vi "FlexMag - 24-03-2023.vi"() -> ()   [LabVIEW 2018] (continued)
                }
              }
              frame True {
                n6892 = stacked-sequence {
                  tunnel: w12617 -> [_ w12620]
                  frame #0 {
                    n6893 = local write "current step"(6.0 ("y")) -> ()
                  }
                  frame #1 {
                    n6894 = Subtract(x=w12620, y=5.0) -> (x-y=w12621:dbl)
                    n6895 = local write "step count"(w12621) -> ()
                  }
                }
              }
            }
            n6896 = local write "QR off mode"(TRUE ("QR manual mode")) -> ()
          }
          frame #1 {
            n6897 = local read "qr wait second"() -> (w12622:u32)
            n6898 = Multiply(x=u32 1000 ("milliseconds to wait"), y=w12622) -> (x*y=w12623:u32)
            n6899 = Wait (ms)(milliseconds to wait=w12623) -> ()  [unwired: 1 out]
          }
          frame #2 {
            n6900 = disable-structure shown="Disabled" {
              frame Disabled {
                n6901 = local write "Interrupt DI"(TRUE ("Interrupt DI")) -> ()
                n6902 = Wait (ms)(milliseconds to wait=u32 100) -> ()  [unwired: 1 out]
              }
              frame Enabled {
              }
            }
          }
          frame #3 {
            n6903 = local read "step count"() -> (w12628:dbl)
            n6904 = Greater?(x=w12628, y=0.0) -> (0:w12629:bool)
            n6905 = case shown="True" w12629 {
              frame False {
              }
              frame True {
                n6906 = local write "QR continuous mode"(TRUE ("QR continuous mode")) -> ()
              }
            }
          }
        }
      }
      frame 7 {
        # "barcode 6"
        n6907 = stacked-sequence {
          frame #0 {
            n6908 = local read "forward roll"() -> (w12633:bool)
            n6909 = local read "step count 2"() -> (w12631:dbl)
            n6910 = local read "back roll"() -> (w12632:bool)
            n6911 = Wait (ms)(milliseconds to wait=u32 100) -> ()  [unwired: 1 out]
            n6912 = case shown="False" w12633 {
              tunnel: w12632 -> [w12636 _]
              tunnel: w12631 -> [_ w12639]
              frame False {
                n6913 = case shown="True" w12636 {
                  frame False {
                  }
                  frame True {
                    n6914 = stacked-sequence {
                      frame #0 {
                        n6915 = local write "current step"(6.0 ("current step")) -> ()
                      }
                      frame #1 {
                        n6916 = local write "step count"(6.0 ("y")) -> ()
                      }
                    }
                  }
                }
              }
              frame True {
                n6917 = stacked-sequence {
                  tunnel: w12639 -> [_ w12642]
                  frame #0 {
                    n6918 = local write "current step"(7.0 ("y")) -> ()
                  }
                  frame #1 {
                    n6919 = Subtract(x=w12642, y=6.0) -> (x-y=w12643:dbl)
                    n6920 = local write "step count"(w12643) -> ()
                  }
                }
              }
            }
            n6921 = local write "QR off mode"(TRUE ("QR manual mode")) -> ()
          }
          frame #1 {
            n6922 = local read "qr wait second"() -> (w12644:u32)
            n6923 = Multiply(x=u32 1000 ("milliseconds to wait"), y=w12644) -> (x*y=w12645:u32)
            n6924 = Wait (ms)(milliseconds to wait=w12645) -> ()  [unwired: 1 out]
          }
          frame #2 {
            n6925 = disable-structure shown="Disabled" {
              frame Disabled {
                n6926 = local write "Interrupt DI"(TRUE ("Interrupt DI")) -> ()
                n6927 = Wait (ms)(milliseconds to wait=u32 100) -> ()  [unwired: 1 out]
              }
              frame Enabled {
              }
            }
          }
          frame #3 {
            n6928 = local read "step count"() -> (w12650:dbl)
            n6929 = Greater?(x=w12650, y=0.0) -> (0:w12651:bool)
            n6930 = case shown="True" w12651 {
              frame False {
              }
              frame True {
                n6931 = local write "QR continuous mode"(TRUE ("QR continuous mode")) -> ()
              }
            }
          }
        }
      }
      frame 8 {
        # "barcode 7"
        n6932 = stacked-sequence {
          frame #0 {
            n6933 = local read "forward roll"() -> (w12655:bool)
            n6934 = local read "step count 2"() -> (w12653:dbl)
            n6935 = local read "back roll"() -> (w12654:bool)
            n6936 = Wait (ms)(milliseconds to wait=u32 100) -> ()  [unwired: 1 out]
            n6937 = case shown="True" w12655 {
              tunnel: w12654 -> [w12658 _]
              tunnel: w12653 -> [_ w12661]
              frame False {
                n6938 = case shown="True" w12658 {
                  frame False {
                  }
                  frame True {
                    n6939 = stacked-sequence {
                      frame #0 {
                        n6940 = local write "current step"(7.0 ("current step")) -> ()
                      }
                      frame #1 {
                        n6941 = local write "step count"(7.0 ("y")) -> ()
                      }
                    }
                  }
                }
              }
              frame True {
                n6942 = stacked-sequence {
                  tunnel: w12661 -> [_ w12664]
                  frame #0 {
                    n6943 = local write "current step"(8.0 ("y")) -> ()
                  }
                  frame #1 {
                    n6944 = Subtract(x=w12664, y=7.0) -> (x-y=w12665:dbl)
                    n6945 = local write "step count"(w12665) -> ()
                  }
                }
              }
            }
            n6946 = local write "QR off mode"(TRUE ("QR manual mode")) -> ()
          }
          frame #1 {
            n6947 = local read "qr wait second"() -> (w12666:u32)
            n6948 = Multiply(x=u32 1000 ("milliseconds to wait"), y=w12666) -> (x*y=w12667:u32)
            n6949 = Wait (ms)(milliseconds to wait=w12667) -> ()  [unwired: 1 out]
          }
          frame #2 {
            n6950 = disable-structure shown="Disabled" {
              frame Disabled {
                n6951 = local write "Interrupt DI"(TRUE ("Interrupt DI")) -> ()
                n6952 = Wait (ms)(milliseconds to wait=u32 100) -> ()  [unwired: 1 out]
              }
              frame Enabled {
              }
            }
          }
          frame #3 {
            n6953 = local read "step count"() -> (w12672:dbl)
            n6954 = Greater?(x=w12672, y=0.0) -> (0:w12673:bool)
            n6955 = case shown="True" w12673 {
              frame False {
              }
              frame True {
                n6956 = local write "QR continuous mode"(TRUE ("QR continuous mode")) -> ()
              }
            }
          }
        }
      }
      frame 9 {
        # "barcode 8"
        n6957 = stacked-sequence {
          frame #0 {
            n6958 = local read "forward roll"() -> (w12677:bool)
            n6959 = local read "step count 2"() -> (w12675:dbl)
            n6960 = local read "back roll"() -> (w12676:bool)
            n6961 = Wait (ms)(milliseconds to wait=u32 100) -> ()  [unwired: 1 out]
            n6962 = case shown="False" w12677 {
              tunnel: w12676 -> [w12680 _]
              tunnel: w12675 -> [_ w12683]
              frame False {
                n6963 = case shown="True" w12680 {
                  frame False {
                  }
                  frame True {
                    n6964 = stacked-sequence {
                      frame #0 {
                        n6965 = local write "current step"(8.0 ("current step")) -> ()
                      }
                      frame #1 {
                        n6966 = local write "step count"(8.0 ("y")) -> ()
                      }
                    }
                  }
                }
              }
              frame True {
                n6967 = stacked-sequence {
                  tunnel: w12683 -> [_ w12686]
                  frame #0 {
                    n6968 = local write "current step"(9.0 ("y")) -> ()
                  }
                  frame #1 {
                    n6969 = Subtract(x=w12686, y=8.0) -> (x-y=w12687:dbl)
                    n6970 = local write "step count"(w12687) -> ()
                  }
                }
              }
            }
            n6971 = local write "QR off mode"(TRUE ("QR manual mode")) -> ()
          }
          frame #1 {
            n6972 = local read "qr wait second"() -> (w12688:u32)
            n6973 = Multiply(x=u32 1000 ("milliseconds to wait"), y=w12688) -> (x*y=w12689:u32)
            n6974 = Wait (ms)(milliseconds to wait=w12689) -> ()  [unwired: 1 out]
          }
          frame #2 {
            n6975 = disable-structure shown="Disabled" {
              frame Disabled {
                n6976 = local write "Interrupt DI"(TRUE ("Interrupt DI")) -> ()
                n6977 = Wait (ms)(milliseconds to wait=u32 100) -> ()  [unwired: 1 out]
              }
              frame Enabled {
              }
            }
          }
          frame #3 {
            n6978 = local read "step count"() -> (w12694:dbl)
            n6979 = Greater?(x=w12694, y=0.0) -> (0:w12695:bool)
            n6980 = case shown="True" w12695 {
              frame False {
              }
              frame True {
                n6981 = local write "QR continuous mode"(TRUE ("QR continuous mode")) -> ()
              }
            }
          }
        }
      }
      frame 10 {
        # "barcode 9"
        n6982 = stacked-sequence {
          frame #0 {
            n6983 = local read "forward roll"() -> (w12699:bool)
            n6984 = local read "step count 2"() -> (w12697:dbl)
            n6985 = local read "back roll"() -> (w12698:bool)
            n6986 = Wait (ms)(milliseconds to wait=u32 100) -> ()  [unwired: 1 out]
            n6987 = case shown="True" w12699 {
              tunnel: w12698 -> [w12702 _]
              tunnel: w12697 -> [_ w12705]
              frame False {
                n6988 = case shown="True" w12702 {
                  frame False {
                  }
                  frame True {
                    n6989 = stacked-sequence {
                      frame #0 {
                        n6990 = local write "current step"(9.0 ("current step")) -> ()
                      }
                      frame #1 {
                        n6991 = local write "step count"(9.0 ("y")) -> ()
                      }
                    }
                  }
                }
              }
              frame True {
                n6992 = stacked-sequence {
                  tunnel: w12705 -> [_ w12708]
                  frame #0 {
                    n6993 = local write "current step"(10.0 ("y")) -> ()
                  }
                  frame #1 {
                    n6994 = Subtract(x=w12708, y=9.0) -> (x-y=w12709:dbl)
                    n6995 = local write "step count"(w12709) -> ()
                  }
                }
              }
            }
            n6996 = local write "QR off mode"(TRUE ("QR manual mode")) -> ()
          }
          frame #1 {
            n6997 = local read "qr wait second"() -> (w12710:u32)
            n6998 = Multiply(x=u32 1000 ("milliseconds to wait"), y=w12710) -> (x*y=w12711:u32)
            n6999 = Wait (ms)(milliseconds to wait=w12711) -> ()  [unwired: 1 out]
          }
          frame #2 {
            n7000 = disable-structure shown="Disabled" {
              frame Disabled {
                n7001 = local write "Interrupt DI"(TRUE ("Interrupt DI")) -> ()
                n7002 = Wait (ms)(milliseconds to wait=u32 100) -> ()  [unwired: 1 out]
              }
              frame Enabled {
              }
            }
          }
          frame #3 {
            n7003 = local read "step count"() -> (w12716:dbl)
            n7004 = Greater?(x=w12716, y=0.0) -> (0:w12717:bool)
            n7005 = case shown="True" w12717 {
              frame False {
              }
              frame True {
                n7006 = local write "QR continuous mode"(TRUE ("QR continuous mode")) -> ()
              }
            }
          }
        }
      }
      frame 11 {
        # "barcode 10"
        n7007 = stacked-sequence {
          frame #0 {
            n7008 = local read "forward roll"() -> (w12721:bool)
            n7009 = local read "step count 2"() -> (w12719:dbl)
            n7010 = local read "back roll"() -> (w12720:bool)
            n7011 = Wait (ms)(milliseconds to wait=u32 100) -> ()  [unwired: 1 out]
            n7012 = case shown="False" w12721 {
              tunnel: w12720 -> [w12724 _]
              tunnel: w12719 -> [_ w12727]
              frame False {
                n7013 = case shown="True" w12724 {
                  frame False {
                  }
                  frame True {
                    n7014 = stacked-sequence {
                      frame #0 {
                        n7015 = local write "current step"(10.0 ("current step")) -> ()
                      }
                      frame #1 {
                        n7016 = local write "step count"(10.0 ("y")) -> ()
                      }
                    }
                  }
                }
              }
              frame True {
                n7017 = stacked-sequence {
                  tunnel: w12727 -> [_ w12730]
                  frame #0 {
                    n7018 = local write "current step"(11.0 ("y")) -> ()
                  }
                  frame #1 {
                    n7019 = Subtract(x=w12730, y=10.0) -> (x-y=w12731:dbl)
                    n7020 = local write "step count"(w12731) -> ()
                  }
                }
              }
            }
            n7021 = local write "QR off mode"(TRUE ("QR manual mode")) -> ()
          }
          frame #1 {
            n7022 = local read "qr wait second"() -> (w12732:u32)
            n7023 = Multiply(x=u32 1000 ("milliseconds to wait"), y=w12732) -> (x*y=w12733:u32)
            n7024 = Wait (ms)(milliseconds to wait=w12733) -> ()  [unwired: 1 out]
          }
          frame #2 {
            n7025 = disable-structure shown="Disabled" {
              frame Disabled {
                n7026 = local write "Interrupt DI"(TRUE ("Interrupt DI")) -> ()
                n7027 = Wait (ms)(milliseconds to wait=u32 100) -> ()  [unwired: 1 out]
              }
              frame Enabled {
              }
            }
          }
          frame #3 {
            n7028 = local read "step count"() -> (w12738:dbl)
            n7029 = Greater?(x=w12738, y=0.0) -> (0:w12739:bool)
            n7030 = case shown="True" w12739 {
              frame False {
              }
              frame True {
                n7031 = local write "QR continuous mode"(TRUE ("QR continuous mode")) -> ()
              }
            }
          }
        }
      }
      frame 12 {
        # "barcode 11"
        n7032 = stacked-sequence {
          frame #0 {
            n7033 = local read "forward roll"() -> (w12743:bool)
            n7034 = local read "step count 2"() -> (w12741:dbl)
            n7035 = local read "back roll"() -> (w12742:bool)
            n7036 = Wait (ms)(milliseconds to wait=u32 100) -> ()  [unwired: 1 out]
            n7037 = case shown="False" w12743 {
              tunnel: w12742 -> [w12746 _]
              tunnel: w12741 -> [_ w12749]
              frame False {
                n7038 = case shown="True" w12746 {
                  frame False {
                  }
                  frame True {
                    n7039 = stacked-sequence {
                      frame #0 {
                        n7040 = local write "current step"(11.0 ("current step")) -> ()
                      }
                      frame #1 {
                        n7041 = local write "step count"(11.0 ("y")) -> ()
                      }
                    }
                  }
                }
              }
              frame True {
                n7042 = stacked-sequence {
                  tunnel: w12749 -> [_ w12752]
                  frame #0 {
                    n7043 = local write "current step"(12.0 ("y")) -> ()
                  }
                  frame #1 {
                    n7044 = Subtract(x=w12752, y=11.0) -> (x-y=w12753:dbl)
                    n7045 = local write "step count"(w12753) -> ()
                  }
                }
              }
            }
            n7046 = local write "QR off mode"(TRUE ("QR manual mode")) -> ()
          }
          frame #1 {
            n7047 = local read "qr wait second"() -> (w12754:u32)
            n7048 = Multiply(x=u32 1000 ("milliseconds to wait"), y=w12754) -> (x*y=w12755:u32)
            n7049 = Wait (ms)(milliseconds to wait=w12755) -> ()  [unwired: 1 out]
          }
          frame #2 {
            n7050 = disable-structure shown="Disabled" {
              frame Disabled {
                n7051 = local write "Interrupt DI"(TRUE ("Interrupt DI")) -> ()
                n7052 = Wait (ms)(milliseconds to wait=u32 100) -> ()  [unwired: 1 out]
              }
              frame Enabled {
              }
            }
          }
          frame #3 {
            n7053 = local read "step count"() -> (w12760:dbl)
            n7054 = Greater?(x=w12760, y=0.0) -> (0:w12761:bool)
            n7055 = case shown="True" w12761 {
              frame False {
              }
              frame True {
                n7056 = local write "QR continuous mode"(TRUE ("QR continuous mode")) -> ()
              }
            }
          }
        }
      }
      frame 13 {
        # "barcode 12"
        n7057 = stacked-sequence {
          frame #0 {
            n7058 = local read "forward roll"() -> (w12765:bool)
            n7059 = local read "step count 2"() -> (w12763:dbl)
            n7060 = local read "back roll"() -> (w12764:bool)
            n7061 = Wait (ms)(milliseconds to wait=u32 100) -> ()  [unwired: 1 out]
            n7062 = case shown="False" w12765 {
              tunnel: w12764 -> [w12768 _]
              tunnel: w12763 -> [_ w12771]
              frame False {
                n7063 = case shown="True" w12768 {
                  frame False {
                  }
                  frame True {
                    n7064 = stacked-sequence {
                      frame #0 {
                        n7065 = local write "current step"(12.0 ("current step")) -> ()
                      }
                      frame #1 {
                        n7066 = local write "step count"(12.0 ("y")) -> ()
                      }
                    }
                  }
                }
              }
              frame True {
                n7067 = stacked-sequence {
                  tunnel: w12771 -> [_ w12774]
                  frame #0 {
                    n7068 = local write "current step"(13.0 ("y")) -> ()
                  }
                  frame #1 {
                    n7069 = Subtract(x=w12774, y=12.0) -> (x-y=w12775:dbl)
                    n7070 = local write "step count"(w12775) -> ()
                  }
                }
              }
            }
            n7071 = local write "QR off mode"(TRUE ("QR manual mode")) -> ()
          }
          frame #1 {
            n7072 = local read "qr wait second"() -> (w12776:u32)
            n7073 = Multiply(x=u32 1000 ("milliseconds to wait"), y=w12776) -> (x*y=w12777:u32)
            n7074 = Wait (ms)(milliseconds to wait=w12777) -> ()  [unwired: 1 out]
          }
          frame #2 {
            n7075 = disable-structure shown="Disabled" {
              frame Disabled {
                n7076 = local write "Interrupt DI"(TRUE ("Interrupt DI")) -> ()
                n7077 = Wait (ms)(milliseconds to wait=u32 100) -> ()  [unwired: 1 out]
              }
              frame Enabled {
              }
            }
          }
          frame #3 {
            n7078 = local read "step count"() -> (w12782:dbl)
            n7079 = Greater?(x=w12782, y=0.0) -> (0:w12783:bool)
            n7080 = case shown="True" w12783 {
              frame False {
              }
              frame True {
                n7081 = local write "QR continuous mode"(TRUE ("QR continuous mode")) -> ()
              }
            }
          }
        }
      }
      frame 14 {
        # "barcode 13"
        n7082 = stacked-sequence {
          frame #0 {
            n7083 = local read "forward roll"() -> (w12787:bool)
            n7084 = local read "step count 2"() -> (w12785:dbl)
            n7085 = local read "back roll"() -> (w12786:bool)
            n7086 = Wait (ms)(milliseconds to wait=u32 100) -> ()  [unwired: 1 out]
            n7087 = case shown="True" w12787 {
              tunnel: w12786 -> [w12790 _]
              tunnel: w12785 -> [_ w12793]
              frame False {
                n7088 = case shown="True" w12790 {
                  frame False {
                  }
                  frame True {
                    n7089 = stacked-sequence {
                      frame #0 {
                        n7090 = local write "current step"(13.0 ("current step")) -> ()
                      }
                      frame #1 {
                        n7091 = local write "step count"(13.0 ("y")) -> ()
                      }
                    }
                  }
                }
              }
              frame True {
                n7092 = stacked-sequence {
                  tunnel: w12793 -> [_ w12796]
                  frame #0 {
                    n7093 = local write "current step"(14.0 ("y")) -> ()
                  }
                  frame #1 {
                    n7094 = Subtract(x=w12796, y=13.0) -> (x-y=w12797:dbl)
                    n7095 = local write "step count"(w12797) -> ()
                  }
                }
              }
            }
            n7096 = local write "QR off mode"(TRUE ("QR manual mode")) -> ()
          }
          frame #1 {
            n7097 = local read "qr wait second"() -> (w12798:u32)
            n7098 = Multiply(x=u32 1000 ("milliseconds to wait"), y=w12798) -> (x*y=w12799:u32)
            n7099 = Wait (ms)(milliseconds to wait=w12799) -> ()  [unwired: 1 out]
          }
          frame #2 {
            n7100 = disable-structure shown="Disabled" {
              frame Disabled {
                n7101 = local write "Interrupt DI"(TRUE ("Interrupt DI")) -> ()
                n7102 = Wait (ms)(milliseconds to wait=u32 100) -> ()  [unwired: 1 out]
              }
              frame Enabled {
              }
            }
          }
          frame #3 {
            n7103 = local read "step count"() -> (w12804:dbl)
            n7104 = Greater?(x=w12804, y=0.0) -> (0:w12805:bool)
            n7105 = case shown="True" w12805 {
              frame False {
              }
              frame True {
                n7106 = local write "QR continuous mode"(TRUE ("QR continuous mode")) -> ()
              }
            }
          }
        }
      }
      frame 15 {
        # "barcode 14"
        n7107 = stacked-sequence {
          frame #0 {
            n7108 = local read "forward roll"() -> (w12809:bool)
            n7109 = local read "step count 2"() -> (w12807:dbl)
            n7110 = local read "back roll"() -> (w12808:bool)
            n7111 = Wait (ms)(milliseconds to wait=u32 100) -> ()  [unwired: 1 out]
            n7112 = case shown="False" w12809 {
              tunnel: w12808 -> [w12812 _]
              tunnel: w12807 -> [_ w12815]
              frame False {
                n7113 = case shown="True" w12812 {
                  frame False {
                  }
                  frame True {
                    n7114 = stacked-sequence {
                      frame #0 {
                        n7115 = local write "current step"(14.0 ("current step")) -> ()
                      }
                      frame #1 {
                        n7116 = local write "step count"(14.0 ("y")) -> ()
                      }
                    }
                  }
                }
              }
              frame True {
                n7117 = stacked-sequence {
                  tunnel: w12815 -> [_ w12818]
                  frame #0 {
                    n7118 = local write "current step"(15.0 ("y")) -> ()
                  }
                  frame #1 {
                    n7119 = Subtract(x=w12818, y=14.0) -> (x-y=w12819:dbl)
                    n7120 = local write "step count"(w12819) -> ()
                  }
                }
              }
            }
            n7121 = local write "QR off mode"(TRUE ("QR manual mode")) -> ()
          }
          frame #1 {
            n7122 = local read "qr wait second"() -> (w12820:u32)
            n7123 = Multiply(x=u32 1000 ("milliseconds to wait"), y=w12820) -> (x*y=w12821:u32)
            n7124 = Wait (ms)(milliseconds to wait=w12821) -> ()  [unwired: 1 out]
          }
          frame #2 {
            n7125 = disable-structure shown="Disabled" {
              frame Disabled {
                n7126 = local write "Interrupt DI"(TRUE ("Interrupt DI")) -> ()
                n7127 = Wait (ms)(milliseconds to wait=u32 100) -> ()  [unwired: 1 out]
              }
              frame Enabled {
              }
            }
          }
          frame #3 {
            n7128 = local read "step count"() -> (w12826:dbl)
            n7129 = Greater?(x=w12826, y=0.0) -> (0:w12827:bool)
            n7130 = case shown="True" w12827 {
              frame False {
              }
              frame True {
                n7131 = local write "QR continuous mode"(TRUE ("QR continuous mode")) -> ()
              }
            }
          }
        }
      }
      frame 16 {
        # "barcode 15"
        n7132 = stacked-sequence {
          frame #0 {
            n7133 = local read "forward roll"() -> (w12831:bool)
            n7134 = local read "step count 2"() -> (w12829:dbl)
            n7135 = local read "back roll"() -> (w12830:bool)
            n7136 = Wait (ms)(milliseconds to wait=u32 100) -> ()  [unwired: 1 out]
            n7137 = case shown="True" w12831 {
              tunnel: w12830 -> [w12834 _]
              tunnel: w12829 -> [_ w12837]
              frame False {
                n7138 = case shown="True" w12834 {
                  frame False {
                  }
                  frame True {
                    n7139 = stacked-sequence {
                      frame #0 {
                        n7140 = local write "current step"(15.0 ("current step")) -> ()
                      }
                      frame #1 {
                        n7141 = local write "step count"(15.0 ("y")) -> ()
                      }
                    }
                  }
                }
              }
              frame True {
                n7142 = stacked-sequence {
                  tunnel: w12837 -> [_ w12840]
                  frame #0 {
                    n7143 = local write "current step"(16.0 ("y")) -> ()
                  }
                  frame #1 {
                    n7144 = Subtract(x=w12840, y=15.0) -> (x-y=w12841:dbl)
                    n7145 = local write "step count"(w12841) -> ()
                  }
                }
              }
            }
            n7146 = local write "QR off mode"(TRUE ("QR manual mode")) -> ()
          }
          frame #1 {
            n7147 = local read "qr wait second"() -> (w12842:u32)
            n7148 = Multiply(x=u32 1000 ("milliseconds to wait"), y=w12842) -> (x*y=w12843:u32)
            n7149 = Wait (ms)(milliseconds to wait=w12843) -> ()  [unwired: 1 out]
          }
          frame #2 {
            n7150 = disable-structure shown="Disabled" {
              frame Disabled {
                n7151 = local write "Interrupt DI"(TRUE ("Interrupt DI")) -> ()
                n7152 = Wait (ms)(milliseconds to wait=u32 100) -> ()  [unwired: 1 out]
              }
              frame Enabled {
              }
            }
          }
          frame #3 {
            n7153 = local read "step count"() -> (w12848:dbl)
            n7154 = Greater?(x=w12848, y=0.0) -> (0:w12849:bool)
            n7155 = case shown="True" w12849 {
              frame False {
              }
              frame True {
                n7156 = local write "QR continuous mode"(TRUE ("QR continuous mode")) -> ()
              }
            }
          }
        }
      }
      frame 17 {
        # "barcode 16"
        n7157 = stacked-sequence {
          frame #0 {
            n7158 = local read "forward roll"() -> (w12853:bool)
            n7159 = local read "step count 2"() -> (w12851:dbl)
            n7160 = local read "back roll"() -> (w12852:bool)
            n7161 = Wait (ms)(milliseconds to wait=u32 100) -> ()  [unwired: 1 out]
            n7162 = case shown="True" w12853 {
              tunnel: w12852 -> [w12856 _]
              tunnel: w12851 -> [_ w12859]
              frame False {
                n7163 = case shown="True" w12856 {
                  frame False {
                  }
                  frame True {
                    n7164 = stacked-sequence {
                      frame #0 {
                        n7165 = local write "current step"(16.0 ("current step")) -> ()
                      }
                      frame #1 {
                        n7166 = local write "step count"(16.0 ("y")) -> ()
                      }
                    }
                  }
                }
              }
              frame True {
                n7167 = stacked-sequence {
                  tunnel: w12859 -> [_ w12862]
                  frame #0 {
                    n7168 = local write "current step"(17.0 ("y")) -> ()
                  }
                  frame #1 {
                    n7169 = Subtract(x=w12862, y=16.0) -> (x-y=w12863:dbl)
                    n7170 = local write "step count"(w12863) -> ()
                  }
                }
              }
            }
            n7171 = local write "QR off mode"(TRUE ("QR manual mode")) -> ()
          }
          frame #1 {
            n7172 = local read "qr wait second"() -> (w12864:u32)
            n7173 = Multiply(x=u32 1000 ("milliseconds to wait"), y=w12864) -> (x*y=w12865:u32)
            n7174 = Wait (ms)(milliseconds to wait=w12865) -> ()  [unwired: 1 out]
          }
          frame #2 {
            n7175 = disable-structure shown="Disabled" {
              frame Disabled {
                n7176 = local write "Interrupt DI"(TRUE ("Interrupt DI")) -> ()
                n7177 = Wait (ms)(milliseconds to wait=u32 100) -> ()  [unwired: 1 out]
              }
              frame Enabled {
              }
            }
          }
          frame #3 {
            n7178 = local read "step count"() -> (w12870:dbl)
            n7179 = Greater?(x=w12870, y=0.0) -> (0:w12871:bool)
            n7180 = case shown="True" w12871 {
              frame False {
              }
              frame True {
                n7181 = local write "QR continuous mode"(TRUE ("QR continuous mode")) -> ()
              }
            }
          }
        }
      }
      frame 18 {
        # "barcode 17"
        n7182 = stacked-sequence {
          frame #0 {
            n7183 = local read "forward roll"() -> (w12875:bool)
            n7184 = local read "step count 2"() -> (w12873:dbl)
            n7185 = local read "back roll"() -> (w12874:bool)
            n7186 = Wait (ms)(milliseconds to wait=u32 100) -> ()  [unwired: 1 out]
            n7187 = case shown="True" w12875 {
              tunnel: w12874 -> [w12878 _]
              tunnel: w12873 -> [_ w12881]
              frame False {
                n7188 = case shown="True" w12878 {
                  frame False {
                  }
                  frame True {
                    n7189 = stacked-sequence {
                      frame #0 {
                        n7190 = local write "current step"(17.0 ("current step")) -> ()
                      }
                      frame #1 {
                        n7191 = local write "step count"(17.0 ("y")) -> ()
                      }
                    }
                  }
                }
              }
              frame True {
                n7192 = stacked-sequence {
                  tunnel: w12881 -> [_ w12884]
                  frame #0 {
                    n7193 = local write "current step"(18.0 ("y")) -> ()
                  }
                  frame #1 {
                    n7194 = Subtract(x=w12884, y=17.0) -> (x-y=w12885:dbl)
                    n7195 = local write "step count"(w12885) -> ()
                  }
                }
              }
            }
            n7196 = local write "QR off mode"(TRUE ("QR manual mode")) -> ()
          }
          frame #1 {
            n7197 = local read "qr wait second"() -> (w12886:u32)
            n7198 = Multiply(x=u32 1000 ("milliseconds to wait"), y=w12886) -> (x*y=w12887:u32)
            n7199 = Wait (ms)(milliseconds to wait=w12887) -> ()  [unwired: 1 out]
          }
          frame #2 {
            n7200 = disable-structure shown="Disabled" {
              frame Disabled {
                n7201 = local write "Interrupt DI"(TRUE ("Interrupt DI")) -> ()
                n7202 = Wait (ms)(milliseconds to wait=u32 100) -> ()  [unwired: 1 out]
              }
              frame Enabled {
              }
            }
          }
          frame #3 {
            n7203 = local read "step count"() -> (w12892:dbl)
            n7204 = Greater?(x=w12892, y=0.0) -> (0:w12893:bool)
            n7205 = case shown="True" w12893 {
              frame False {
              }
              frame True {
                n7206 = local write "QR continuous mode"(TRUE ("QR continuous mode")) -> ()
              }
            }
          }
        }
      }
      frame 19 {
        # "barcode 18"
        n7207 = stacked-sequence {
          frame #0 {
            n7208 = local read "forward roll"() -> (w12897:bool)
            n7209 = local read "step count 2"() -> (w12895:dbl)
            n7210 = local read "back roll"() -> (w12896:bool)
            n7211 = Wait (ms)(milliseconds to wait=u32 100) -> ()  [unwired: 1 out]
            n7212 = case shown="True" w12897 {
              tunnel: w12896 -> [w12900 _]
              tunnel: w12895 -> [_ w12903]
              frame False {
                n7213 = case shown="True" w12900 {
                  frame False {
                  }
                  frame True {
                    n7214 = stacked-sequence {
                      frame #0 {
                        n7215 = local write "current step"(18.0 ("current step")) -> ()
                      }
                      frame #1 {
                        n7216 = local write "step count"(18.0 ("y")) -> ()
                      }
                    }
                  }
                }
              }
              frame True {
                n7217 = stacked-sequence {
                  tunnel: w12903 -> [_ w12906]
                  frame #0 {
                    n7218 = local write "current step"(19.0 ("y")) -> ()
                  }
                  frame #1 {
                    n7219 = Subtract(x=w12906, y=18.0) -> (x-y=w12907:dbl)
                    n7220 = local write "step count"(w12907) -> ()
                  }
                }
              }
            }
            n7221 = local write "QR off mode"(TRUE ("QR manual mode")) -> ()
          }
          frame #1 {
            n7222 = local read "qr wait second"() -> (w12908:u32)
            n7223 = Multiply(x=u32 1000 ("milliseconds to wait"), y=w12908) -> (x*y=w12909:u32)
            n7224 = Wait (ms)(milliseconds to wait=w12909) -> ()  [unwired: 1 out]
          }
          frame #2 {
            n7225 = disable-structure shown="Disabled" {
              frame Disabled {
                n7226 = local write "Interrupt DI"(TRUE ("Interrupt DI")) -> ()
                n7227 = Wait (ms)(milliseconds to wait=u32 100) -> ()  [unwired: 1 out]
              }
              frame Enabled {
              }
            }
          }
          frame #3 {
            n7228 = local read "step count"() -> (w12914:dbl)
            n7229 = Greater?(x=w12914, y=0.0) -> (0:w12915:bool)
            n7230 = case shown="True" w12915 {
              frame False {
              }
              frame True {
                n7231 = local write "QR continuous mode"(TRUE ("QR continuous mode")) -> ()
              }
            }
          }
        }
      }
      frame 20 {
        # "barcode 19"
        n7232 = stacked-sequence {
          frame #0 {
            n7233 = local read "forward roll"() -> (w12919:bool)
            n7234 = local read "step count 2"() -> (w12917:dbl)
            n7235 = local read "back roll"() -> (w12918:bool)
            n7236 = Wait (ms)(milliseconds to wait=u32 100) -> ()  [unwired: 1 out]
            n7237 = case shown="True" w12919 {
              tunnel: w12918 -> [w12922 _]
              tunnel: w12917 -> [_ w12925]
              frame False {
                n7238 = case shown="True" w12922 {
                  frame False {
                  }
                  frame True {
                    n7239 = stacked-sequence {
                      frame #0 {
                        n7240 = local write "current step"(19.0 ("current step")) -> ()
                      }
                      frame #1 {
                        n7241 = local write "step count"(19.0 ("y")) -> ()
                      }
                    }
                  }
                }
              }
              frame True {
                n7242 = stacked-sequence {
                  tunnel: w12925 -> [_ w12928]
                  frame #0 {
                    n7243 = local write "current step"(20.0 ("y")) -> ()
                  }
                  frame #1 {
                    n7244 = Subtract(x=w12928, y=19.0) -> (x-y=w12929:dbl)
                    n7245 = local write "step count"(w12929) -> ()
                  }
                }
              }
            }
            n7246 = local write "QR off mode"(TRUE ("QR manual mode")) -> ()
          }
          frame #1 {
            n7247 = local read "qr wait second"() -> (w12930:u32)
            n7248 = Multiply(x=u32 1000 ("milliseconds to wait"), y=w12930) -> (x*y=w12931:u32)
            n7249 = Wait (ms)(milliseconds to wait=w12931) -> ()  [unwired: 1 out]
          }
          frame #2 {
            n7250 = disable-structure shown="Disabled" {
              frame Disabled {
                n7251 = local write "Interrupt DI"(TRUE ("Interrupt DI")) -> ()
                n7252 = Wait (ms)(milliseconds to wait=u32 100) -> ()  [unwired: 1 out]
              }
              frame Enabled {
              }
            }
          }
          frame #3 {
            n7253 = local read "step count"() -> (w12936:dbl)
            n7254 = Greater?(x=w12936, y=0.0) -> (0:w12937:bool)
            n7255 = case shown="True" w12937 {
              frame False {
              }
              frame True {
                n7256 = local write "QR continuous mode"(TRUE ("QR continuous mode")) -> ()
              }
            }
          }
        }
      }
      frame 21 {
        # "barcode 20"
        n7257 = stacked-sequence {
          frame #0 {
            n7258 = local read "forward roll"() -> (w12941:bool)
            n7259 = local read "step count 2"() -> (w12939:dbl)
            n7260 = local read "back roll"() -> (w12940:bool)
            n7261 = Wait (ms)(milliseconds to wait=u32 100) -> ()  [unwired: 1 out]
            n7262 = case shown="True" w12941 {
              tunnel: w12940 -> [w12944 _]
              tunnel: w12939 -> [_ w12947]
              frame False {
                n7263 = case shown="True" w12944 {
                  frame False {
                  }
                  frame True {
                    n7264 = stacked-sequence {
                      frame #0 {
                        n7265 = local write "current step"(20.0 ("current step")) -> ()
                      }
                      frame #1 {
                        n7266 = local write "step count"(20.0 ("y")) -> ()
                      }
                    }
                  }
                }
              }
              frame True {
                n7267 = stacked-sequence {
                  tunnel: w12947 -> [_ w12950]
                  frame #0 {
                    n7268 = local write "current step"(21.0 ("y")) -> ()
                  }
                  frame #1 {
                    n7269 = Subtract(x=w12950, y=20.0) -> (x-y=w12951:dbl)
                    n7270 = local write "step count"(w12951) -> ()
                  }
                }
              }
            }
            n7271 = local write "QR off mode"(TRUE ("QR manual mode")) -> ()
          }
          frame #1 {
            n7272 = local read "qr wait second"() -> (w12952:u32)
            n7273 = Multiply(x=u32 1000 ("milliseconds to wait"), y=w12952) -> (x*y=w12953:u32)
            n7274 = Wait (ms)(milliseconds to wait=w12953) -> ()  [unwired: 1 out]
          }
          frame #2 {
            n7275 = disable-structure shown="Disabled" {
              frame Disabled {
                n7276 = local write "Interrupt DI"(TRUE ("Interrupt DI")) -> ()
                n7277 = Wait (ms)(milliseconds to wait=u32 100) -> ()  [unwired: 1 out]
              }
              frame Enabled {
              }
            }
          }
          frame #3 {
            n7278 = local read "step count"() -> (w12958:dbl)
            n7279 = Greater?(x=w12958, y=0.0) -> (0:w12959:bool)
            n7280 = case shown="True" w12959 {
              frame False {
              }
              frame True {
                n7281 = local write "QR continuous mode"(TRUE ("QR continuous mode")) -> ()
              }
            }
          }
        }
      }
    }
  }
  n7282 = VISA Close(VISA resource name=w16, error in (no error)=w17) -> ()  [unwired: 1 out]
  n7283 = VISA Close(VISA resource name=w124, error in (no error)=w123) -> ()  [unwired: 1 out]
  n7284 = VISA Close(VISA resource name=w142, error in (no error)=w141) -> ()  [unwired: 1 out]
  n7285 = VISA Close(VISA resource name=w132, error in (no error)=w133) -> ()  [unwired: 1 out]
  n7286 = VISA Close(VISA resource name=w121, error in (no error)=w122) -> ()  [unwired: 1 out]
  n7287 = VISA Close(VISA resource name=w106, error in (no error)=w105) -> ()  [unwired: 1 out]
  n7288 = while {
    stop <- FALSE stop-if-true
    n7289 = stacked-sequence {
      frame #0 {
        n7290 = local read "resolution"() -> (w13148:dbl)
        n7291 = local read "resolution"() -> (w13180:dbl)
        n7292 = local read "CH2_Ai_Ch_Cc"() -> (w13147:u16)
        n7293 = local read "CH2_Ai_Pl_Pg"() -> (w13150:u16)
        n7294 = local read "CH2_Ai_Ch_Pg"() -> (w13149:u16)
        n7295 = local read "CH1_Ai_Ch_Cc"() -> (w13181:u16)
        n7296 = local read "CH1_Ai_Pl_Pg"() -> (w13178:u16)
        n7297 = local read "CH1_Ai_Ch_Pg"() -> (w13179:u16)
        n7298 = Multiply(x=w13148, y=w13150) -> (x*y=w13128:dbl)
        n7299 = Multiply(x=w13148, y=w13147) -> (x*y=w13118:dbl)
        n7300 = Multiply(x=w13148, y=w13149) -> (x*y=w13099:dbl)
        n7301 = Multiply(x=w13180, y=w13178) -> (x*y=w13201:dbl)
        n7302 = Multiply(x=w13180, y=w13179) -> (x*y=w13182:dbl)
        n7303 = Multiply(x=w13180, y=w13181) -> (x*y=w13211:dbl)
        n7304 = feedback #187() -> (w13119:dbl)  [unwired: 1 in]
        n7305 = feedback-in #187(w13118) -> ()
        n7306 = feedback #188() -> (w13129:dbl)  [unwired: 1 in]
        n7307 = feedback-in #188(w13128) -> ()
        n7308 = feedback #189() -> (w13146:dbl)  [unwired: 1 in]
        n7309 = feedback-in #189(w13099) -> ()
        n7310 = feedback #190() -> (w13200:dbl)  [unwired: 1 in]
        n7311 = feedback-in #190(w13201) -> ()
        n7312 = feedback #191() -> (w13183:dbl)  [unwired: 1 in]
        n7313 = feedback-in #191(w13182) -> ()
        n7314 = feedback #192() -> (w13210:dbl)  [unwired: 1 in]
        n7315 = feedback-in #192(w13211) -> ()
        n7316 = feedback #193() -> (w13120:dbl)  [unwired: 1 in]
        n7317 = feedback-in #193(w13119) -> ()
        n7318 = feedback #194() -> (w13130:dbl)  [unwired: 1 in]
        n7319 = feedback-in #194(w13129) -> ()
        n7320 = feedback #195() -> (w13145:dbl)  [unwired: 1 in]
        n7321 = feedback-in #195(w13146) -> ()
        n7322 = feedback #196() -> (w13199:dbl)  [unwired: 1 in]
        n7323 = feedback-in #196(w13200) -> ()
        n7324 = feedback #197() -> (w13184:dbl)  [unwired: 1 in]
        n7325 = feedback-in #197(w13183) -> ()
        n7326 = feedback #198() -> (w13209:dbl)  [unwired: 1 in]
        n7327 = feedback-in #198(w13210) -> ()
        n7328 = feedback #199() -> (w13121:dbl)  [unwired: 1 in]
        n7329 = feedback-in #199(w13120) -> ()
        n7330 = feedback #200() -> (w13131:dbl)  [unwired: 1 in]
        n7331 = feedback-in #200(w13130) -> ()
        n7332 = feedback #201() -> (w13144:dbl)  [unwired: 1 in]
        n7333 = feedback-in #201(w13145) -> ()
        n7334 = feedback #202() -> (w13198:dbl)  [unwired: 1 in]
        n7335 = feedback-in #202(w13199) -> ()
        n7336 = feedback #203() -> (w13185:dbl)  [unwired: 1 in]
        n7337 = feedback-in #203(w13184) -> ()
        n7338 = feedback #204() -> (w13208:dbl)  [unwired: 1 in]
        n7339 = feedback-in #204(w13209) -> ()
        n7340 = feedback #205() -> (w13122:dbl)  [unwired: 1 in]
        n7341 = feedback-in #205(w13121) -> ()
        n7342 = feedback #206() -> (w13132:dbl)  [unwired: 1 in]
        n7343 = feedback-in #206(w13131) -> ()
        n7344 = feedback #207() -> (w13143:dbl)  [unwired: 1 in]
        n7345 = feedback-in #207(w13144) -> ()
        n7346 = feedback #208() -> (w13197:dbl)  [unwired: 1 in]
        n7347 = feedback-in #208(w13198) -> ()
        n7348 = feedback #209() -> (w13186:dbl)  [unwired: 1 in]
        n7349 = feedback-in #209(w13185) -> ()
        n7350 = feedback #210() -> (w13207:dbl)  [unwired: 1 in]
        n7351 = feedback-in #210(w13208) -> ()
        n7352 = feedback #211() -> (w13123:dbl)  [unwired: 1 in]
        n7353 = feedback-in #211(w13122) -> ()
        n7354 = feedback #212() -> (w13133:dbl)  [unwired: 1 in]
        n7355 = feedback-in #212(w13132) -> ()
        n7356 = feedback #213() -> (w13142:dbl)  [unwired: 1 in]
        n7357 = feedback-in #213(w13143) -> ()
        n7358 = feedback #214() -> (w13196:dbl)  [unwired: 1 in]
        n7359 = feedback-in #214(w13197) -> ()
        n7360 = feedback #215() -> (w13187:dbl)  [unwired: 1 in]
        n7361 = feedback-in #215(w13186) -> ()
        n7362 = feedback #216() -> (w13206:dbl)  [unwired: 1 in]
        n7363 = feedback-in #216(w13207) -> ()
        n7364 = feedback #217() -> (w13124:dbl)  [unwired: 1 in]
        n7365 = feedback-in #217(w13123) -> ()
        n7366 = feedback #218() -> (w13134:dbl)  [unwired: 1 in]
        n7367 = feedback-in #218(w13133) -> ()
        n7368 = feedback #219() -> (w13141:dbl)  [unwired: 1 in]
        n7369 = feedback-in #219(w13142) -> ()
        n7370 = feedback #220() -> (w13195:dbl)  [unwired: 1 in]
        n7371 = feedback-in #220(w13196) -> ()
        n7372 = feedback #221() -> (w13188:dbl)  [unwired: 1 in]
        n7373 = feedback-in #221(w13187) -> ()
        n7374 = feedback #222() -> (w13205:dbl)  [unwired: 1 in]
        n7375 = feedback-in #222(w13206) -> ()
        n7376 = feedback #223() -> (w13125:dbl)  [unwired: 1 in]
        n7377 = feedback-in #223(w13124) -> ()
        n7378 = feedback #224() -> (w13135:dbl)  [unwired: 1 in]
        n7379 = feedback-in #224(w13134) -> ()
        n7380 = feedback #225() -> (w13140:dbl)  [unwired: 1 in]
        n7381 = feedback-in #225(w13141) -> ()
        n7382 = feedback #226() -> (w13194:dbl)  [unwired: 1 in]
        n7383 = feedback-in #226(w13195) -> ()
        n7384 = feedback #227() -> (w13189:dbl)  [unwired: 1 in]
        n7385 = feedback-in #227(w13188) -> ()
        n7386 = feedback #228() -> (w13204:dbl)  [unwired: 1 in]
        n7387 = feedback-in #228(w13205) -> ()
        n7388 = feedback #229() -> (w13126:dbl)  [unwired: 1 in]
        n7389 = feedback-in #229(w13125) -> ()
        n7390 = feedback #230() -> (w13136:dbl)  [unwired: 1 in]
        n7391 = feedback-in #230(w13135) -> ()
        n7392 = feedback #231() -> (w13139:dbl)  [unwired: 1 in]
        n7393 = feedback-in #231(w13140) -> ()
        n7394 = feedback #232() -> (w13193:dbl)  [unwired: 1 in]
        n7395 = feedback-in #232(w13194) -> ()
        n7396 = feedback #233() -> (w13190:dbl)  [unwired: 1 in]
        n7397 = feedback-in #233(w13189) -> ()
        n7398 = feedback #234() -> (w13203:dbl)  [unwired: 1 in]
        n7399 = feedback-in #234(w13204) -> ()
        n7400 = feedback #235() -> (w13127:dbl)  [unwired: 1 in]
        n7401 = feedback-in #235(w13126) -> ()
        n7402 = feedback #236() -> (w13137:dbl)  [unwired: 1 in]
        n7403 = feedback-in #236(w13136) -> ()
        n7404 = feedback #237() -> (w13138:dbl)  [unwired: 1 in]
        n7405 = feedback-in #237(w13139) -> ()
        n7406 = feedback #238() -> (w13192:dbl)  [unwired: 1 in]
        n7407 = feedback-in #238(w13193) -> ()
        n7408 = feedback #239() -> (w13191:dbl)  [unwired: 1 in]
        n7409 = feedback-in #239(w13190) -> ()
        n7410 = feedback #240() -> (w13202:dbl)  [unwired: 1 in]
        n7411 = feedback-in #240(w13203) -> ()
        n7412 = Compound Arithmetic op=ADD(w13118, w13119, w13120, w13121, w13122, w13123, w13124, w13125, w13126, w13127) -> (w13115:dbl)
        n7413 = Compound Arithmetic op=ADD(w13128, w13129, w13130, w13131, w13132, w13133, w13134, w13135, w13136, w13137) -> (w13116:dbl)
        n7414 = Compound Arithmetic op=ADD(w13099, w13146, w13145, w13144, w13143, w13142, w13141, w13140, w13139, w13138) -> (w13117:dbl)
        n7415 = Compound Arithmetic op=ADD(w13201, w13200, w13199, w13198, w13197, w13196, w13195, w13194, w13193, w13192) -> (w13213:dbl)
        n7416 = Compound Arithmetic op=ADD(w13182, w13183, w13184, w13185, w13186, w13187, w13188, w13189, w13190, w13191) -> (w13212:dbl)
        n7417 = Compound Arithmetic op=ADD(w13211, w13210, w13209, w13208, w13207, w13206, w13205, w13204, w13203, w13202) -> (w13214:dbl)
        n7418 = Divide(x=w13115, y=10.0) -> (x/y=w13162:dbl)
        "ch2 cc ai(V)" <- w13162
        n7419 = Divide(x=w13116, y=10.0) -> (x/y=w13154:dbl)
        "ch2 pl pg ai(V)" <- w13154
        n7420 = Divide(x=w13117, y=10.0) -> (x/y=w13158:dbl)
        "ch2 ch pg ai(V)" <- w13158
        n7421 = Divide(x=w13213, y=10.0) -> (x/y=w13218:dbl)
        "ch1 pl pg ai(V)" <- w13218
        n7422 = Divide(x=w13212, y=10.0) -> (x/y=w13222:dbl)
        "ch1 ch pg ai(V)" <- w13222
        n7423 = Divide(x=w13214, y=10.0) -> (x/y=w13226:dbl)
        "ch1 cc ai(V)" <- w13226
        n7424 = Subtract(x=w13154, y=5.625) -> (x-y=w13152:dbl)
        n7425 = Subtract(x=w13158, y=5.625) -> (x-y=w13156:dbl)
        n7426 = Subtract(x=w13222, y=5.625) -> (x-y=w13220:dbl)
        n7427 = Subtract(x=w13218, y=5.625) -> (x-y=w13216:dbl)
        n7428 = Subtract(x=w13162, y=10.625) -> (x-y=w13160:dbl)
        n7429 = Power Of 10(x=w13152) -> (10^x=w13151:dbl)
        n7430 = Power Of 10(x=w13156) -> (10^x=w13157:dbl)
        n7431 = Power Of 10(x=w13220) -> (10^x=w13219:dbl)
        n7432 = Subtract(x=w13226, y=10.625) -> (x-y=w13224:dbl)
        n7433 = Power Of 10(x=w13160) -> (10^x=w13159:dbl)
        n7434 = Power Of 10(x=w13216) -> (10^x=w13217:dbl)
        n7435 = In Range and Coerce(upper limit=760.0, x=w13151, lower limit=0.000375) -> (coerced(x)=w13153:dbl)  [unwired: 1 out]
        "ch2 pl pg  torr" <- w13153
        n7436 = In Range and Coerce(upper limit=760.0, x=w13157, lower limit=0.000375) -> (coerced(x)=w13155:dbl)  [unwired: 1 out]
        "ch2 ch pg torr" <- w13155
        n7437 = In Range and Coerce(upper limit=760.0, x=w13219, lower limit=0.000375) -> (coerced(x)=w13221:dbl)  [unwired: 1 out]
        "ch1 ch pg torr" <- w13221
        n7438 = Power Of 10(x=w13224) -> (10^x=w13225:dbl)
        n7439 = In Range and Coerce(upper limit=1.0, x=w13159, lower limit=1e-09) -> (coerced(x)=w13161:dbl)  [unwired: 1 out]
        "ch2 cc torr" <- w13161
        n7440 = In Range and Coerce(upper limit=760.0, x=w13217, lower limit=0.000375) -> (coerced(x)=w13215:dbl)  [unwired: 1 out]
        "ch1 pl pg  torr" <- w13215
        n7441 = Multiply(x=w13153, y=1.33) -> (x*y=w13081:dbl)
        "ch2 pl pg mbar" <- w13081
        "ch2 pl pg mbar gui" <- w13081
        "ch2 pl pg mbar gui 1" <- w13081
        n7442 = In Range and Coerce(upper limit=1.0, x=w13225, lower limit=1e-09) -> (coerced(x)=w13223:dbl)  [unwired: 1 out]
        "ch1 cc torr" <- w13223
        n7443 = Multiply(x=w13155, y=1.33) -> (x*y=w13082:dbl)
        "ch2 ch pg mbar" <- w13082
        "ch2 ch pg mbar gui" <- w13082
        "ch2 ch pg mbar gui 1" <- w13082
        n7444 = Multiply(x=w13221, y=1.33) -> (x*y=w13092:dbl)
        "ch1 ch pg mbar" <- w13092
        "ch1 ch pg mbar gui" <- w13092
        "ch1 ch pg mbar gui 1" <- w13092
        n7445 = Multiply(x=w13161, y=1.33) -> (x*y=w13083:dbl)
        "ch2 cc mbar" <- w13083
        "ch2 cc mbar gui" <- w13083
        "ch2 cc mbar gui 1" <- w13083
        n7446 = Multiply(x=w13215, y=1.33) -> (x*y=w13098:dbl)
        "ch1 pl pg mbar" <- w13098
        "ch1 pl pg mbar gui" <- w13098
        "ch1 pl pg mbar gui 1" <- w13098
        n7447 = Multiply(x=w13223, y=1.33) -> (x*y=w13093:dbl)
        "ch1 cc mbar" <- w13093
        "ch1 cc mbar gui" <- w13093
        "ch1 cc mbar gui 1" <- w13093
        n7448 = Number To Exponential String(number=w13092, precision (6)=i16 3) -> (E-format string=→"CH1 CH PG":string)  [unwired: 2 in]
        n7449 = Number To Exponential String(number=w13093, precision (6)=i16 3) -> (E-format string=→"CH1 CH CC":string)  [unwired: 2 in]
        n7450 = Number To Exponential String(number=w13098, precision (6)=i16 3) -> (E-format string=→"CH1 PL PG":string)  [unwired: 2 in]
        n7451 = Number To Exponential String(number=w13082, precision (6)=i16 3) -> (E-format string=→"CH2 CH PG":string)  [unwired: 2 in]
        n7452 = Number To Exponential String(number=w13083, precision (6)=i16 3) -> (E-format string=→"CH2 CH CC":string)  [unwired: 2 in]
        n7453 = Number To Exponential String(number=w13081, precision (6)=i16 3) -> (E-format string=→"CH2 PL PG":string)  [unwired: 2 in]
      }
      frame #1 {
        n7454 = local read "resolution"() -> (w13274:dbl)
        n7455 = local read "resolution"() -> (w13326:dbl)
        n7456 = local read "CH4_Ai_Ch_Cc"() -> (w13275:u16)
        n7457 = local read "CH4_Ai_Pl_Pg"() -> (w13272:u16)
        n7458 = local read "CH3_Ai_Ch_Cc"() -> (w13327:u16)
        n7459 = local read "CH4_Ai_Ch_Pg"() -> (w13273:u16)
        n7460 = local read "CH3_Ai_Pl_Pg"() -> (w13324:u16)
        n7461 = local read "CH3_Ai_Ch_Pg"() -> (w13325:u16)
        n7462 = Multiply(x=w13274, y=w13272) -> (x*y=w13295:dbl)
        n7463 = Multiply(x=w13274, y=w13275) -> (x*y=w13305:dbl)
        n7464 = Multiply(x=w13274, y=w13273) -> (x*y=w13276:dbl)
        n7465 = Multiply(x=w13326, y=w13324) -> (x*y=w13347:dbl)
        n7466 = Multiply(x=w13326, y=w13327) -> (x*y=w13357:dbl)
        n7467 = Multiply(x=w13326, y=w13325) -> (x*y=w13328:dbl)
        n7468 = feedback #241() -> (w13304:dbl)  [unwired: 1 in]
        n7469 = feedback-in #241(w13305) -> ()
        n7470 = feedback #242() -> (w13294:dbl)  [unwired: 1 in]
        n7471 = feedback-in #242(w13295) -> ()
        n7472 = feedback #243() -> (w13277:dbl)  [unwired: 1 in]
        n7473 = feedback-in #243(w13276) -> ()
        n7474 = feedback #244() -> (w13356:dbl)  [unwired: 1 in]
        n7475 = feedback-in #244(w13357) -> ()
        n7476 = feedback #245() -> (w13346:dbl)  [unwired: 1 in]
        n7477 = feedback-in #245(w13347) -> ()
        n7478 = feedback #246() -> (w13329:dbl)  [unwired: 1 in]
        n7479 = feedback-in #246(w13328) -> ()
        n7480 = feedback #247() -> (w13303:dbl)  [unwired: 1 in]
        n7481 = feedback-in #247(w13304) -> ()
        n7482 = feedback #248() -> (w13293:dbl)  [unwired: 1 in]
        n7483 = feedback-in #248(w13294) -> ()
        n7484 = feedback #249() -> (w13278:dbl)  [unwired: 1 in]
        n7485 = feedback-in #249(w13277) -> ()
        n7486 = feedback #250() -> (w13355:dbl)  [unwired: 1 in]
        n7487 = feedback-in #250(w13356) -> ()
        n7488 = feedback #251() -> (w13345:dbl)  [unwired: 1 in]
        n7489 = feedback-in #251(w13346) -> ()
        n7490 = feedback #252() -> (w13330:dbl)  [unwired: 1 in]
        n7491 = feedback-in #252(w13329) -> ()
        n7492 = feedback #253() -> (w13302:dbl)  [unwired: 1 in]
        n7493 = feedback-in #253(w13303) -> ()
        n7494 = feedback #254() -> (w13292:dbl)  [unwired: 1 in]
        n7495 = feedback-in #254(w13293) -> ()
        n7496 = feedback #255() -> (w13279:dbl)  [unwired: 1 in]
        n7497 = feedback-in #255(w13278) -> ()